vi "Dresden R2R Sputter 03.02.2018 IY24.vi"() -> ()   [LabVIEW 2009] (continued)
                        }
                      }
                      n10678 = Or(x=w17426, y=w17430) -> (x .or. y?=w17427:bool)
                    }
                  }
                  frame #5 {
                    n10679 = local write "Test_stop"(TRUE ("Test_stop")) -> ()
                    n10680 = Wait (ms)(milliseconds to wait=u32 10) -> ()  [unwired: 1 out]
                  }
                }
              }
              frame #1 {
                n10681 = stacked-sequence {
                  tunnel: w17459 -> [_ _ _ _ w17470 _]
                  frame #0 {
                    n10682 = local read "Output voltage value"() -> (w17460:dbl)
                    n10683 = local write "Ch3_SRV_counterclockwise_direction_do"(FALSE ("Ch2_SRV1_direction_do")) -> ()
                    n10684 = local write "Actual Lap"(0.0 ("Actual Lap")) -> ()
                    n10685 = local write "Actual Length"(0.0 ("Actual Region")) -> ()
                    n10686 = Wait (ms)(milliseconds to wait=u32 10) -> ()  [unwired: 1 out]
                    n10687 = local write "Tension_controller1_set_value"(w17460) -> ()
                  }
                  frame #1 {
                    n10688 = local write "Tension_controller1_set"(TRUE ("Tension_controller2_set")) -> ()
                  }
                  frame #2 {
                    n10689 = Wait (ms)(milliseconds to wait=u32 10) -> ()  [unwired: 1 out]
                  }
                  frame #3 {
                    n10690 = local write "Tension_controllers_start/stop_do"(TRUE ("Tension_controllers_start/stop_do")) -> ()
                    n10691 = local write "Ch3_SRV_start_stop_do"(TRUE ("Ch2_SRV1_start_stop_do")) -> ()
                    n10692 = Wait (ms)(milliseconds to wait=u32 10) -> ()  [unwired: 1 out]
                  }
                  frame #4 {
                    n10693 = while {
                      tunnel: w17470 -> [w17472]
                      stop <- w17474 stop-if-true
                      n10694 = Wait Until Next ms Multiple(millisecond multiple=u32 10) -> ()  [unwired: 1 out]
                      n10695 = call "Elapsed Time153"("Reset"=w17472) -> ("Elapsed Time (s)"=w17476:dbl)  [unwired: 11 in, 7 out]
                      "Elapsed Time (s) 10" <- w17476
                      n10696 = case shown="True" FALSE {
                        frame #0 {
                          n10697 = local read "To Left Volt"() -> (w17481:dbl)
                          n10698 = local write "Tension_controller1_set"(TRUE ("Tension_controller2_set")) -> ()
                          n10699 = local write "Tension_controller1_set_value"(w17481) -> ()
                        }
                        frame #1 {
                          n10700 = stacked-sequence {
                            frame #0 {
                              n10701 = local read "Actual Diameter"() -> (w17489:dbl)
                              n10702 = local read "Actual Diameter"() -> (w17486:dbl)
                              n10703 = local read "Web Thickness"() -> (w17495:dbl)
                              n10704 = local read "Actual Lap"() -> (w17487:dbl)
                              n10705 = Increment(x=w17487) -> (x+1=w17485:dbl)
                              n10706 = local read "Actual Length"() -> (w17488:dbl)
                              n10707 = Multiply(x=w17495, y=0.002) -> (x*y=w17496:dbl)
                              n10708 = Multiply(x=w17489, y=3.14) -> (x*y=w17491:dbl)
                              n10709 = local write "Actual Lap"(w17485) -> ()
                              n10710 = Add(x=w17486, y=w17496) -> (x+y=w17494:dbl)
                              n10711 = Divide(x=w17491, y=1000.0) -> (x/y=w17493:dbl)
                              n10712 = local write "Actual Diameter"(w17494) -> ()
                              n10713 = Add(x=w17493, y=w17488) -> (x+y=w17484:dbl)
                              n10714 = disable-structure shown="Disabled" {
                                frame #0 {
                                n10715 = local read "Output voltage value"() -> (w17500:dbl)
                                n10716 = local read "Set voltage value"() -> (w17499:dbl)
                                n10717 = Subtract(x=w17500, y=w17499) -> (x-y=w17498:dbl)
                                n10718 = local write "Output voltage value"(w17498) -> ()
                                }
                                frame #1 {
                                }
                              }
                              n10719 = local write "Actual Length"(w17484) -> ()
                              n10720 = Wait (ms)(milliseconds to wait=u32 10) -> ()  [unwired: 1 out]
                            }
                            frame #1 {
                              n10721 = local read "Output voltage value"() -> (w17501:dbl)
                              n10722 = local write "Tension_controller1_set_value"(w17501) -> ()
                              n10723 = Wait (ms)(milliseconds to wait=u32 10) -> ()  [unwired: 1 out]
                            }
                            frame #2 {
                              n10724 = local write "Tension_controller1_set"(TRUE ("Tension_controller2_set")) -> ()
                              "Actual Region led 5" <- TRUE ("Actual Region")
                            }
                          }
                        }
                      }
                      n10725 = Greater Or Equal?(x=w17476, y="Right to Left 5") -> (x >= y?=w17473:bool)
                      n10726 = local read "Start_roll"() -> (w17479:bool)
                      n10727 = Not(x=w17479) -> (.not. x?=w17477:bool)
                      n10728 = Or(x=w17473, y=w17477) -> (x .or. y?=w17474:bool)
                      n10729 = case shown="True" w17473 {
                        frame #0 {
                        }
                        frame #1 {
                          n10730 = local write "Ch3_SRV_start_stop_do"(FALSE ("Ch2_SRV1_start_stop_do")) -> ()
                        }
                      }
                    }
                  }
                  frame #5 {
                    n10731 = local write "Test_stop"(TRUE ("Test_stop")) -> ()
                    n10732 = Wait (ms)(milliseconds to wait=u32 10) -> ()  [unwired: 1 out]
                  }
                }
              }
            }
          }
          frame #4 {
            n10733 = local read "Roll_side_select"() -> (w17508:enum32{"Left to Right", "Right to Left"})
            n10734 = case shown="\"Left to Right\", Default" w17508 {
              tunnel: w17507 -> [_ w17556]
              tunnel: w17507 -> [w17509 _]
              frame #0 {
                n10735 = stacked-sequence {
                  tunnel: w17509 -> [_ _ _ _ w17520 _]
                  frame #0 {
                    n10736 = local read "Output voltage value"() -> (w17512:dbl)
                    n10737 = local write "Ch4_SRV_counterclockwise_direction_do"(TRUE ("Ch2_SRV1_direction_do")) -> ()
                    n10738 = local write "Actual Lap"(0.0 ("Actual Lap")) -> ()
                    n10739 = local write "Actual Length"(0.0 ("Actual Region")) -> ()
                    n10740 = Wait (ms)(milliseconds to wait=u32 10) -> ()  [unwired: 1 out]
                    n10741 = local write "Tension_controller2_set_value"(w17512) -> ()
                  }
                  frame #1 {
                    n10742 = local write "Tension_controller2_set"(TRUE ("Tension_controller2_set")) -> ()
                  }
                  frame #2 {
                    n10743 = Wait (ms)(milliseconds to wait=u32 10) -> ()  [unwired: 1 out]
                  }
                  frame #3 {
                    n10744 = local write "Tension_controllers_start/stop_do"(TRUE ("Tension_controllers_start/stop_do")) -> ()
                    n10745 = local write "Ch4_SRV_start_stop_do"(TRUE ("Ch2_SRV1_start_stop_do")) -> ()
                    n10746 = Wait (ms)(milliseconds to wait=u32 10) -> ()  [unwired: 1 out]
                  }
                  frame #4 {
                    n10747 = while {
                      tunnel: w17520 -> [w17522]
                      stop <- w17524 stop-if-true
                      n10748 = call "Elapsed Time147"("Reset"=w17522) -> ("Elapsed Time (s)"=w17526:dbl)  [unwired: 11 in, 7 out]
                      "Elapsed Time (s) 7" <- w17526
                      n10749 = Wait Until Next ms Multiple(millisecond multiple=u32 10) -> ()  [unwired: 1 out]
                      n10750 = local read "Start_roll"() -> (w17529:bool)
                      n10751 = Greater Or Equal?(x=w17526, y="Left to Right 4") -> (x >= y?=w17523:bool)
                      n10752 = case shown="True" FALSE {
                        frame #0 {
                          n10753 = local read "To Right Volt"() -> (w17531:dbl)
                          n10754 = local write "Tension_controller2_set_value"(w17531) -> ()
                          n10755 = local write "Tension_controller2_set"(TRUE ("Tension_controller2_set")) -> ()
                        }
                        frame #1 {
                          n10756 = stacked-sequence {
                            frame #0 {
                              n10757 = local read "Actual Diameter"() -> (w17538:dbl)
                              n10758 = local read "Web Thickness"() -> (w17545:dbl)
                              n10759 = local read "Actual Diameter"() -> (w17539:dbl)
                              n10760 = local read "Actual Lap"() -> (w17533:dbl)
                              n10761 = Multiply(x=w17545, y=0.002) -> (x*y=w17546:dbl)
                              n10762 = Increment(x=w17533) -> (x+1=w17534:dbl)
                              n10763 = Add(x=w17538, y=w17546) -> (x+y=w17544:dbl)
                              n10764 = local read "Actual Length"() -> (w17535:dbl)
                              n10765 = Multiply(x=w17539, y=3.14) -> (x*y=w17541:dbl)
                              n10766 = local write "Actual Diameter"(w17544) -> ()
                              n10767 = local write "Actual Lap"(w17534) -> ()
                              n10768 = Divide(x=w17541, y=1000.0) -> (x/y=w17543:dbl)
                              n10769 = Add(x=w17543, y=w17535) -> (x+y=w17536:dbl)
                              n10770 = disable-structure shown="Disabled" {
                                frame #0 {
                                n10771 = local read "Output voltage value"() -> (w17550:dbl)
                                n10772 = local read "Set voltage value"() -> (w17549:dbl)
                                n10773 = Subtract(x=w17550, y=w17549) -> (x-y=w17548:dbl)
                                n10774 = local write "Output voltage value"(w17548) -> ()
                                }
                                frame #1 {
                                }
                              }
                              n10775 = Wait (ms)(milliseconds to wait=u32 10) -> ()  [unwired: 1 out]
                              n10776 = local write "Actual Length"(w17536) -> ()
                            }
                            frame #1 {
                              n10777 = local read "Output voltage value"() -> (w17551:dbl)
                              n10778 = Wait (ms)(milliseconds to wait=u32 10) -> ()  [unwired: 1 out]
                              n10779 = local write "Tension_controller2_set_value"(w17551) -> ()
                            }
                            frame #2 {
                              n10780 = local write "Tension_controller2_set"(TRUE ("Tension_controller2_set")) -> ()
                            }
                          }
                        }
                      }
                      n10781 = Not(x=w17529) -> (.not. x?=w17527:bool)
                      n10782 = case shown="True" w17523 {
                        frame #0 {
                        }
                        frame #1 {
                          n10783 = local write "Ch4_SRV_start_stop_do"(FALSE ("Ch2_SRV1_start_stop_do")) -> ()
                        }
                      }
                      n10784 = Or(x=w17523, y=w17527) -> (x .or. y?=w17524:bool)
                    }
                  }
                  frame #5 {
                    n10785 = local write "Test_stop"(TRUE ("Test_stop")) -> ()
                    n10786 = Wait (ms)(milliseconds to wait=u32 10) -> ()  [unwired: 1 out]
                  }
                }
              }
              frame #1 {
                n10787 = stacked-sequence {
                  tunnel: w17556 -> [_ _ _ _ w17567 _]
                  frame #0 {
                    n10788 = local read "Output voltage value"() -> (w17557:dbl)
                    n10789 = local write "Ch4_SRV_counterclockwise_direction_do"(FALSE ("Ch2_SRV1_direction_do")) -> ()
                    n10790 = local write "Actual Lap"(0.0 ("Actual Lap")) -> ()
                    n10791 = local write "Actual Length"(0.0 ("Actual Region")) -> ()
                    n10792 = Wait (ms)(milliseconds to wait=u32 10) -> ()  [unwired: 1 out]
                    n10793 = local write "Tension_controller1_set_value"(w17557) -> ()
                  }
                  frame #1 {
                    n10794 = local write "Tension_controller1_set"(TRUE ("Tension_controller2_set")) -> ()
                  }
                  frame #2 {
                    n10795 = Wait (ms)(milliseconds to wait=u32 10) -> ()  [unwired: 1 out]
                  }
                  frame #3 {
                    n10796 = local write "Tension_controllers_start/stop_do"(TRUE ("Tension_controllers_start/stop_do")) -> ()
                    n10797 = local write "Ch4_SRV_start_stop_do"(TRUE ("Ch2_SRV1_start_stop_do")) -> ()
                    n10798 = Wait (ms)(milliseconds to wait=u32 10) -> ()  [unwired: 1 out]
                  }
                  frame #4 {
                    n10799 = while {
                      tunnel: w17567 -> [w17569]
                      stop <- w17571 stop-if-true
                      n10800 = Wait Until Next ms Multiple(millisecond multiple=u32 10) -> ()  [unwired: 1 out]
                      n10801 = call "Elapsed Time148"("Reset"=w17569) -> ("Elapsed Time (s)"=w17573:dbl)  [unwired: 11 in, 7 out]
                      "Elapsed Time (s) 8" <- w17573
                      n10802 = case shown="True" FALSE {
                        frame #0 {
                          n10803 = local read "To Left Volt"() -> (w17578:dbl)
                          n10804 = local write "Tension_controller1_set"(TRUE ("Tension_controller2_set")) -> ()
                          n10805 = local write "Tension_controller1_set_value"(w17578) -> ()
                        }
                        frame #1 {
                          n10806 = stacked-sequence {
                            frame #0 {
                              n10807 = local read "Actual Diameter"() -> (w17586:dbl)
                              n10808 = local read "Actual Diameter"() -> (w17583:dbl)
                              n10809 = local read "Web Thickness"() -> (w17592:dbl)
                              n10810 = local read "Actual Lap"() -> (w17584:dbl)
                              n10811 = Increment(x=w17584) -> (x+1=w17582:dbl)
                              n10812 = local read "Actual Length"() -> (w17585:dbl)
                              n10813 = Multiply(x=w17592, y=0.002) -> (x*y=w17593:dbl)
                              n10814 = Multiply(x=w17586, y=3.14) -> (x*y=w17588:dbl)
                              n10815 = local write "Actual Lap"(w17582) -> ()
                              n10816 = Add(x=w17583, y=w17593) -> (x+y=w17591:dbl)
                              n10817 = Divide(x=w17588, y=1000.0) -> (x/y=w17590:dbl)
                              n10818 = local write "Actual Diameter"(w17591) -> ()
                              n10819 = Add(x=w17590, y=w17585) -> (x+y=w17581:dbl)
                              n10820 = disable-structure shown="Disabled" {
                                frame #0 {
                                n10821 = local read "Output voltage value"() -> (w17597:dbl)
                                n10822 = local read "Set voltage value"() -> (w17596:dbl)
                                n10823 = Subtract(x=w17597, y=w17596) -> (x-y=w17595:dbl)
                                n10824 = local write "Output voltage value"(w17595) -> ()
                                }
                                frame #1 {
                                }
                              }
                              n10825 = local write "Actual Length"(w17581) -> ()
                              n10826 = Wait (ms)(milliseconds to wait=u32 10) -> ()  [unwired: 1 out]
                            }
                            frame #1 {
                              n10827 = local read "Output voltage value"() -> (w17598:dbl)
                              n10828 = local write "Tension_controller1_set_value"(w17598) -> ()
                              n10829 = Wait (ms)(milliseconds to wait=u32 10) -> ()  [unwired: 1 out]
                            }
                            frame #2 {
                              n10830 = local write "Tension_controller1_set"(TRUE ("Tension_controller2_set")) -> ()
                              "Actual Region led 4" <- TRUE ("Actual Region")
                            }
                          }
                        }
                      }
                      n10831 = Greater Or Equal?(x=w17573, y="Right to Left 4") -> (x >= y?=w17570:bool)
                      n10832 = local read "Start_roll"() -> (w17576:bool)
                      n10833 = Not(x=w17576) -> (.not. x?=w17574:bool)
                      n10834 = Or(x=w17570, y=w17574) -> (x .or. y?=w17571:bool)
                      n10835 = case shown="True" w17570 {
                        frame #0 {
                        }
                        frame #1 {
                          n10836 = local write "Ch4_SRV_start_stop_do"(FALSE ("Ch2_SRV1_start_stop_do")) -> ()
                        }
                      }
                    }
                  }
                  frame #5 {
                    n10837 = local write "Test_stop"(TRUE ("Test_stop")) -> ()
                    n10838 = Wait (ms)(milliseconds to wait=u32 10) -> ()  [unwired: 1 out]
                  }
                }
              }
            }
          }
        }
      }
    }
  }
  n10839 = while {
    stop <- FALSE stop-if-true
    n10840 = Wait Until Next ms Multiple(millisecond multiple=u32 300) -> ()  [unwired: 1 out]
    n10841 = case shown="True" "Automatic Roll" {
      tunnel: "Auto_roll_ch_select" -> [_ w17608]
      frame #0 {
      }
      frame #1 {
        n10842 = stacked-sequence {
          tunnel: w17608 -> [_ _ _ _ _ w17629 _ _ _ _ _ _ _ _ _ _ _]
          frame #0 {
            n10843 = local write "Calculate_auto"(TRUE ("Calculate_auto")) -> ()
            n10844 = Wait (ms)(milliseconds to wait=u32 100) -> ()  [unwired: 1 out]
          }
          frame #1 {
            n10845 = while {
              stop <- w17611 stop-if-true
              n10846 = local read "Automatic Roll"() -> (w17614:bool)
              n10847 = local read "Calculate_auto"() -> (w17616:bool)
              n10848 = Wait Until Next ms Multiple(millisecond multiple=u32 100 ("milliseconds to wait")) -> ()  [unwired: 1 out]
              n10849 = local read "Semi"() -> (w17612:bool)
              n10850 = Not(x=w17614) -> (.not. x?=w17613:bool)
              n10851 = Not(x=w17616) -> (.not. x?=w17615:bool)
              n10852 = Compound Arithmetic op=OR(w17615, w17613, w17612) -> (w17611:bool)
            }
          }
          frame #2 {
            n10853 = local write "Roll_side_select"(enum32{"Left to Right", "Right to Left"}."Left to Right" ("Roll_side_select")) -> ()
            n10854 = Wait (ms)(milliseconds to wait=u32 100) -> ()  [unwired: 1 out]
          }
          frame #3 {
            n10855 = Wait (ms)(milliseconds to wait=u32 100) -> ()  [unwired: 1 out]
            n10856 = local write "Parameters_auto_set"(TRUE ("Calculate_auto")) -> ()
          }
          frame #4 {
            n10857 = while {
              stop <- w17622 stop-if-true
              n10858 = local read "Parameters_auto_set"() -> (w17627:bool)
              n10859 = local read "Automatic Roll"() -> (w17625:bool)
              n10860 = Wait Until Next ms Multiple(millisecond multiple=u32 100 ("milliseconds to wait")) -> ()  [unwired: 1 out]
              n10861 = local read "Semi"() -> (w17623:bool)
              n10862 = Not(x=w17625) -> (.not. x?=w17624:bool)
              n10863 = Not(x=w17627) -> (.not. x?=w17626:bool)
              n10864 = Compound Arithmetic op=OR(w17626, w17624, w17623) -> (w17622:bool)
            }
          }
          frame #5 {
            n10865 = local write "Target Chamber Sensor"(w17629) -> ()
            n10866 = Wait (ms)(milliseconds to wait=u32 100) -> ()  [unwired: 1 out]
          }
          frame #6 {
            n10867 = Wait (ms)(milliseconds to wait=u32 100) -> ()  [unwired: 1 out]
            n10868 = local write "Start_roll"(TRUE ("Calculate_auto")) -> ()
          }
          frame #7 {
            n10869 = while {
              stop <- w17633 stop-if-true
              n10870 = local read "Start_roll"() -> (w17638:bool)
              n10871 = local read "Automatic Roll"() -> (w17636:bool)
              n10872 = Wait Until Next ms Multiple(millisecond multiple=u32 100 ("milliseconds to wait")) -> ()  [unwired: 1 out]
              n10873 = local read "Semi"() -> (w17634:bool)
              n10874 = Not(x=w17636) -> (.not. x?=w17635:bool)
              n10875 = Not(x=w17638) -> (.not. x?=w17637:bool)
              n10876 = Compound Arithmetic op=OR(w17637, w17635, w17634) -> (w17633:bool)
            }
          }
          frame #8 {
            n10877 = Wait (ms)(milliseconds to wait=u32 2500) -> ()  [unwired: 1 out]
          }
          frame #9 {
            n10878 = local write "Calculate_auto"(TRUE ("Calculate_auto")) -> ()
            n10879 = Wait (ms)(milliseconds to wait=u32 100) -> ()  [unwired: 1 out]
          }
          frame #10 {
            n10880 = while {
              stop <- w17643 stop-if-true
              n10881 = local read "Automatic Roll"() -> (w17646:bool)
              n10882 = local read "Calculate_auto"() -> (w17648:bool)
              n10883 = Wait Until Next ms Multiple(millisecond multiple=u32 100 ("milliseconds to wait")) -> ()  [unwired: 1 out]
              n10884 = local read "Semi"() -> (w17644:bool)
              n10885 = Not(x=w17646) -> (.not. x?=w17645:bool)
              n10886 = Not(x=w17648) -> (.not. x?=w17647:bool)
              n10887 = Compound Arithmetic op=OR(w17647, w17645, w17644) -> (w17643:bool)
            }
          }
          frame #11 {
            n10888 = local write "Roll_side_select"(enum32{"Left to Right", "Right to Left"}."Right to Left" ("Roll_side_select")) -> ()
            n10889 = Wait (ms)(milliseconds to wait=u32 100) -> ()  [unwired: 1 out]
          }
          frame #12 {
            n10890 = Wait (ms)(milliseconds to wait=u32 100) -> ()  [unwired: 1 out]
            n10891 = local write "Parameters_auto_set"(TRUE ("Calculate_auto")) -> ()
          }
          frame #13 {
            n10892 = while {
              stop <- w17654 stop-if-true
              n10893 = local read "Parameters_auto_set"() -> (w17659:bool)
              n10894 = local read "Automatic Roll"() -> (w17657:bool)
              n10895 = Wait Until Next ms Multiple(millisecond multiple=u32 100 ("milliseconds to wait")) -> ()  [unwired: 1 out]
              n10896 = local read "Semi"() -> (w17655:bool)
              n10897 = Not(x=w17657) -> (.not. x?=w17656:bool)
              n10898 = Not(x=w17659) -> (.not. x?=w17658:bool)
              n10899 = Compound Arithmetic op=OR(w17658, w17656, w17655) -> (w17654:bool)
            }
          }
          frame #14 {
            n10900 = Wait (ms)(milliseconds to wait=u32 100) -> ()  [unwired: 1 out]
            n10901 = local write "Start_roll"(TRUE ("Calculate_auto")) -> ()
          }
          frame #15 {
            n10902 = while {
              stop <- w17663 stop-if-true
              n10903 = local read "Start_roll"() -> (w17668:bool)
              n10904 = local read "Automatic Roll"() -> (w17666:bool)
              n10905 = Wait Until Next ms Multiple(millisecond multiple=u32 100 ("milliseconds to wait")) -> ()  [unwired: 1 out]
              n10906 = local read "Semi"() -> (w17664:bool)
              n10907 = Not(x=w17666) -> (.not. x?=w17665:bool)
              n10908 = Not(x=w17668) -> (.not. x?=w17667:bool)
              n10909 = Compound Arithmetic op=OR(w17667, w17665, w17664) -> (w17663:bool)
            }
          }
          frame #16 {
            n10910 = local read "Auto_roll_completed_cycle"() -> (w17671:dbl)
            n10911 = Increment(x=w17671) -> (x+1=w17670:dbl)
            n10912 = Wait (ms)(milliseconds to wait=u32 2500) -> ()  [unwired: 1 out]
            n10913 = local write "Auto_roll_completed_cycle"(w17670) -> ()
          }
        }
      }
    }
  }
  n10914 = VISA Close(VISA resource name=w798, error in (no error)=w799) -> ()  [unwired: 1 out]
  n10915 = VISA Close(VISA resource name=w811, error in (no error)=w810) -> ()  [unwired: 1 out]
  n10916 = while {
    stop <- i16? 0 stop-if-true
    # "TP STATUTE"
    n10917 = stacked-sequence {
      frame #0 {
        n10918 = local read "after substring"() -> (w17678)
        n10919 = local read "Tp1_speed_gui"() -> (w17675)
        n10920 = String Length(string=w17678) -> (length=w17681)
        n10921 = Not Equal To 0?(x=w17681) -> (x != 0?=w17679)
        n10922 = Greater?(x=w17675, y="Tp_max_speed") -> (0:w17677)
        n10923 = case shown="False" w17677 {
          tunnel: [w17684 "Maximum Speed" ("Tp1_statute 2")] -> w17676
          tunnel: w17679 -> [w17683 _]
          tunnel: w17678 -> [w17682 _]
          frame #0 {
            n10924 = case shown="True" w17683 {
              tunnel: [" No connection!" ("Tp1_statute 2") w17688] -> w17684
              tunnel: w17682 -> [_ w17687]
              frame #0 {
                n10925 = local write "Ch1_Tp_on"(i16? 0 ("Tp_on(ch1)")) -> ()
              }
              frame #1 {
                n10926 = String Subset(string=w17687, length (rest)=i32? 6 ("length (rest)")) -> (substring=w17692)  [unwired: 1 out]
                n10927 = Equal?(x=w17692, y="000000") -> (x = y?=w17689)
                n10928 = case shown="True" w17689 {
                  tunnel: ["Accelarating" ("Tp1_statute 2") w17695] -> w17688
                  frame #0 {
                    w17693 = T/1 ("Tp1_accelarate")
                    n10929 = local write "Ch1_Tp_on"(w17693) -> ()
                    "Tp1_accelarate" <- w17693
                  }
                  frame #1 {
                    n10930 = local read "Tp1_speed_gui"() -> (w17696)
                    n10931 = Equal?(x=w17696, y=data[9B]) -> (x = y?=w17698)
                    n10932 = case shown="False" w17698 {
                      tunnel: ["Decelarating" ("Tp1_statute 2") "Stopped" ("Tp1_statute 2")] -> w17695
                      frame #0 {
                        n10933 = local write "Ch1_Tp_on"(i16? 0 ("Tp_on(ch1)")) -> ()
                        "Tp1_decelarate" <- T/1 ("Tp1_decelarate")
                      }
                      frame #1 {
                        n10934 = local write "Ch1_Tp_on"(i16? 0 ("Tp_on(ch1)")) -> ()
                      }
                    }
                  }
                }
              }
            }
          }
          frame #1 {
            n10935 = local write "Ch1_Tp_on"(T/1 ("Tp1_accelarate")) -> ()
          }
        }
        "Tp1_statute" <- w17676
      }
      frame #1 {
        n10936 = local read "Tp2_speed_gui"() -> (w17706)
        n10937 = local read "after substring 2"() -> (w17709)
        n10938 = String Length(string=w17709) -> (length=w17712)
        n10939 = Not Equal To 0?(x=w17712) -> (x != 0?=w17710)
        n10940 = Greater?(x=w17706, y="Tp2_max_speed") -> (0:w17708)
        n10941 = case shown="False" w17708 {
          tunnel: [w17715 "Maximum Speed" ("Tp1_statute 2")] -> w17707
          tunnel: w17710 -> [w17714 _]
          tunnel: w17709 -> [w17713 _]
          frame #0 {
            n10942 = case shown="True" w17714 {
              tunnel: [" No connection!" ("Tp1_statute 2") w17719] -> w17715
              tunnel: w17713 -> [_ w17718]
              frame #0 {
                n10943 = local write "Ch2_Tp_on"(i16? 0 ("Tp_on(ch1)")) -> ()
              }
              frame #1 {
                n10944 = String Subset(string=w17718, length (rest)=i32? 6 ("length (rest)")) -> (substring=w17723)  [unwired: 1 out]
                n10945 = Equal?(x=w17723, y="000000") -> (x = y?=w17720)
                n10946 = case shown="True" w17720 {
                  tunnel: ["Accelarating" ("Tp1_statute 2") w17726] -> w17719
                  frame #0 {
                    w17724 = T/1 ("Tp1_accelarate")
                    n10947 = local write "Ch2_Tp_on"(w17724) -> ()
                    "Tp2_accelarate" <- w17724
                  }
                  frame #1 {
                    n10948 = local read "Tp2_speed_gui"() -> (w17728)
                    n10949 = Equal?(x=w17728, y=data[9B]) -> (x = y?=w17727)
                    n10950 = case shown="False" w17727 {
                      tunnel: ["Decelarating" ("Tp1_statute 2") "Stopped" ("Tp1_statute 2")] -> w17726
                      frame #0 {
                        n10951 = local write "Ch2_Tp_on"(i16? 0 ("Tp_on(ch1)")) -> ()
                        "Tp2_decelarate" <- T/1 ("Tp1_decelarate")
                      }
                      frame #1 {
                        n10952 = local write "Ch2_Tp_on"(i16? 0 ("Tp_on(ch1)")) -> ()
                      }
                    }
                  }
                }
              }
            }
          }
          frame #1 {
            n10953 = local write "Ch2_Tp_on"(T/1 ("Tp_on(ch1)")) -> ()
          }
        }
        "Tp2_statute" <- w17707
      }
      frame #2 {
        n10954 = local read "after substring 3"() -> (w17741)
        n10955 = local read "Tp3_speed_gui"() -> (w17737)
        n10956 = String Length(string=w17741) -> (length=w17743)
        n10957 = Not Equal To 0?(x=w17743) -> (x != 0?=w17742)
        n10958 = Greater?(x=w17737, y="Tp3_max_speed") -> (0:w17740)
        n10959 = case shown="False" w17740 {
          tunnel: [w17746 "Maximum Speed" ("Tp1_statute 2")] -> w17739
          tunnel: w17742 -> [w17745 _]
          tunnel: w17741 -> [w17744 _]
          frame #0 {
            n10960 = case shown="True" w17745 {
              tunnel: [" No connection!" ("Tp1_statute 2") w17750] -> w17746
              tunnel: w17744 -> [_ w17749]
              frame #0 {
                n10961 = local write "Ch3_Tp_on"(i16? 0 ("Tp_on(ch1)")) -> ()
              }
              frame #1 {
                n10962 = String Subset(string=w17749, length (rest)=i32? 6 ("length (rest)")) -> (substring=w17754)  [unwired: 1 out]
                n10963 = Equal?(x=w17754, y="000000") -> (x = y?=w17751)
                n10964 = case shown="True" w17751 {
                  tunnel: ["Accelarating" ("Tp1_statute 2") w17757] -> w17750
                  frame #0 {
                    w17755 = T/1 ("Tp1_accelarate")
                    n10965 = local write "Ch3_Tp_on"(w17755) -> ()
                    "Tp3_accelarate" <- w17755
                  }
                  frame #1 {
                    n10966 = local read "Tp3_speed_gui"() -> (w17759)
                    n10967 = Equal?(x=w17759, y=data[9B]) -> (x = y?=w17758)
                    n10968 = case shown="False" w17758 {
                      tunnel: ["Decelarating" ("Tp1_statute 2") "Stopped" ("Tp1_statute 2")] -> w17757
                      frame #0 {
                        n10969 = local write "Ch3_Tp_on"(i16? 0 ("Tp_on(ch1)")) -> ()
                        "Tp3_decelarate" <- T/1 ("Tp1_decelarate")
                      }
                      frame #1 {
                        n10970 = local write "Ch3_Tp_on"(i16? 0 ("Tp_on(ch1)")) -> ()
                      }
                    }
                  }
                }
              }
            }
          }
          frame #1 {
            n10971 = local write "Ch3_Tp_on"(T/1 ("Tp1_accelarate")) -> ()
          }
        }
        "Tp3_statute" <- w17739
      }
      frame #3 {
        n10972 = local read "Turbo_pump_speed 4"() -> (w17772)
        n10973 = local read "after substring 4"() -> (w17770)
        n10974 = String Length(string=w17770) -> (length=w17774)
        n10975 = Not Equal To 0?(x=w17774) -> (x != 0?=w17771)
        n10976 = Greater?(x=w17772, y="Tp4_max_speed") -> (0:w17769)
        n10977 = case shown="False" w17769 {
          tunnel: [w17777 "Maximum Speed" ("Tp1_statute 2")] -> w17768
          tunnel: w17771 -> [w17776 _]
          tunnel: w17770 -> [w17775 _]
          frame #0 {
            n10978 = case shown="True" w17776 {
              tunnel: [" No connection!" ("Tp1_statute 2") w17781] -> w17777
              tunnel: w17775 -> [_ w17780]
              frame #0 {
                n10979 = local write "Ch4_Tp_on"(i16? 0 ("Tp_on(ch1)")) -> ()
              }
              frame #1 {
                n10980 = String Subset(string=w17780, length (rest)=i32? 6 ("length (rest)")) -> (substring=w17785)  [unwired: 1 out]
                n10981 = Equal?(x=w17785, y="000000") -> (x = y?=w17782)
                n10982 = case shown="False" w17782 {
                  tunnel: ["Accelarating" ("Tp1_statute 2") w17789] -> w17781
                  frame #0 {
                    n10983 = local write "Ch4_Tp_on"(T/1 ("Tp_on(ch1)")) -> ()
                    "Tp4_accelarate" <- T/1 ("Tp1_accelarate")
                  }
                  frame #1 {
                    n10984 = local read "Tp4_speed_gui"() -> (w17791)
                    n10985 = Equal?(x=w17791, y=data[9B]) -> (x = y?=w17790)
                    n10986 = case shown="False" w17790 {
                      tunnel: ["Decelarating" ("Tp1_statute 2") "Stopped" ("Tp1_statute 2")] -> w17789
                      frame #0 {
                        n10987 = local write "Ch4_Tp_on"(i16? 0 ("Tp_on(ch1)")) -> ()
                        "Tp4_decelarate" <- T/1 ("Tp1_decelarate")
                      }
                      frame #1 {
                        n10988 = local write "Ch4_Tp_on"(i16? 0 ("Tp_on(ch1)")) -> ()
                      }
                    }
                  }
                }
              }
            }
          }
          frame #1 {
            n10989 = local write "Ch4_Tp_on"(T/1 ("Tp1_accelarate")) -> ()
          }
        }
        "Tp4_statute" <- w17768
      }
    }
    n10990 = Wait Until Next ms Multiple(millisecond multiple=i32? 300) -> ()  [unwired: 1 out]
  }
  n10991 = VISA Close(VISA resource name=w25, error in (no error)=w24) -> ()  [unwired: 1 out]
  n10992 = VISA Close(VISA resource name=w735, error in (no error)=w734) -> ()  [unwired: 1 out]
  n10993 = VISA Close(VISA resource name=w802, error in (no error)=w801) -> ()  [unwired: 1 out]
  n10994 = VISA Close(VISA resource name=w808, error in (no error)=w807) -> ()  [unwired: 1 out]
  n10995 = VISA Close(VISA resource name=w782, error in (no error)=w781) -> ()  [unwired: 1 out]
  n10996 = while {
    stop <- i16? 0 stop-if-true
    n10997 = local read "Tp1_stop_cmnd"() -> (w17833)
    n10998 = local read "Tp2_stop_cmnd"() -> (w17823)
    n10999 = local read "Tp3_stop_cmnd"() -> (w17815)
    n11000 = local read "Tp4_stop_cmnd"() -> (w17809)
    n11001 = local read "Tp3_statute"() -> (w17801)
    n11002 = Wait Until Next ms Multiple(millisecond multiple=i32? 300) -> ()  [unwired: 1 out]
    n11003 = local read "Tp2_statute"() -> (w17817)
    n11004 = local read "Tp1_statute"() -> (w17824)
    n11005 = local read "Tp4_statute"() -> (w17800)
    n11006 = case shown="True" w17833 {
      tunnel: [w17856 i16? 0] -> w17832
      frame #0 {
        n11007 = local read "Tp1_statute"() -> (w17855)
        n11008 = Equal?(x="Accelarating", y=w17855) -> (x = y?=w17860)
        n11009 = Equal?(x=w17855, y="Maximum Speed") -> (x = y?=w17859)
        n11010 = Or(x=w17860, y=w17859) -> (x .or. y?=w17856)
      }
      frame #1 {
      }
    }
    "TP1_working" <- w17832
    n11011 = Equal?(x="Decelarating", y=w17817) -> (x = y?=w17821)
    n11012 = Equal?(x=w17817, y="Stopped") -> (x = y?=w17816)
    n11013 = case shown="False" w17823 {
      tunnel: [w17849 i16? 0] -> w17822
      frame #0 {
        n11014 = local read "Tp2_statute"() -> (w17848)
        n11015 = Equal?(x="Accelarating", y=w17848) -> (x = y?=w17853)
        n11016 = Equal?(x=w17848, y="Maximum Speed") -> (x = y?=w17852)
        n11017 = Or(x=w17853, y=w17852) -> (x .or. y?=w17849)
      }
      frame #1 {
      }
    }
    "TP2_working" <- w17822
    n11018 = case shown="True" w17815 {
      tunnel: [w17842 i16? 0] -> w17808
      frame #0 {
        n11019 = local read "Tp3_statute"() -> (w17841)
        n11020 = Equal?(x="Accelarating", y=w17841) -> (x = y?=w17846)
        n11021 = Equal?(x=w17841, y="Maximum Speed") -> (x = y?=w17845)
        n11022 = Or(x=w17846, y=w17845) -> (x .or. y?=w17842)
      }
      frame #1 {
      }
    }
    "TP3_working" <- w17808
    n11023 = case shown="False" w17809 {
      tunnel: [w17835 i16? 0] -> w17807
      frame #0 {
        n11024 = local read "Tp4_statute"() -> (w17834)
        n11025 = Equal?(x="Accelarating", y=w17834) -> (x = y?=w17839)
        n11026 = Equal?(x=w17834, y="Maximum Speed") -> (x = y?=w17838)
        n11027 = Or(x=w17839, y=w17838) -> (x .or. y?=w17835)
      }
      frame #1 {
      }
    }
    "TP4_working" <- w17807
    n11028 = Equal?(x="Decelarating", y=w17824) -> (x = y?=w17828)
    n11029 = Equal?(x=w17824, y="Stopped") -> (x = y?=w17829)
    n11030 = Equal?(x="Decelarating", y=w17800) -> (x = y?=w17806)
    n11031 = Equal?(x=w17800, y="Stopped") -> (x = y?=w17805)
    n11032 = Equal?(x="Decelarating", y=w17801) -> (x = y?=w17811)
    n11033 = Equal?(x=w17801, y="Stopped") -> (x = y?=w17812)
    n11034 = Or(x=w17821, y=w17816) -> (x .or. y?=→"Tp2_stopped")
    n11035 = Or(x=w17828, y=w17829) -> (x .or. y?=→"Tp1_stopped")
    n11036 = Or(x=w17806, y=w17805) -> (x .or. y?=→"Tp4_stopped")
    n11037 = Or(x=w17811, y=w17812) -> (x .or. y?=→"Tp3_stopped")
  }
  n11038 = VISA Close(VISA resource name=w743, error in (no error)=w774) -> ()  [unwired: 1 out]
  n11039 = VISA Close(VISA resource name=w744, error in (no error)=w759) -> ()  [unwired: 1 out]
  n11040 = VISA Close(VISA resource name=w757, error in (no error)=w758) -> ()  [unwired: 1 out]
  n11041 = VISA Close(VISA resource name=w745, error in (no error)=w773) -> ()  [unwired: 1 out]
  n11042 = while {
    stop <- FALSE stop-if-true
    n11043 = Wait Until Next ms Multiple(millisecond multiple=u32 300) -> ()  [unwired: 1 out]
    n11044 = Build Array(FALSE, "Transfer_ch1_2", "Transfer_ch2_1", "Transfer_ch2_3", "Transfer_ch3_2", "Transfer_ch3_4", "Transfer_ch4_3") -> (w17870:bool[])
    n11045 = Boolean Array To Number(Boolean array=w17870) -> (number=w17871:u32)
    n11046 = Mantissa & Exponent(0:w17871) -> (2:w17868:dbl)  [unwired: 1 out]
    n11047 = case shown="1" w17868 {
      frame #0 {
      }
      frame #1 {
        n11048 = stacked-sequence {
          frame #0 {
            n11049 = Wait (ms)(milliseconds to wait=u32 1500) -> ()  [unwired: 1 out]
            n11050 = local write "Clean_trnsfr_1_2"(TRUE ("Clean_trnsfr_1_2")) -> ()
            n11051 = local write "system_status"("Chamber 1 to Chamber 2 Transfer Process in Progress." ("system_status")) -> ()
            n11052 = local write "final_process_messages"("Chamber 1 to Chamber 2  Transfer Process was completed." ("final_process_messages")) -> ()
          }
          frame #1 {
            n11053 = stacked-sequence {
              frame #0 {
                n11054 = local write "Routine_check_transfer"(TRUE ("Routine_check_transfer")) -> ()
                n11055 = Wait (ms)(milliseconds to wait=u32 100) -> ()  [unwired: 1 out]
              }
              frame #1 {
                n11056 = while {
                  i -> [w17887]
                  stop <- w17883 stop-if-true
                  n11057 = Greater Or Equal?(x=w17887, y=1500) -> (x >= y?=w17884:bool)
                  n11058 = Wait Until Next ms Multiple(millisecond multiple=u32 200) -> ()  [unwired: 1 out]
                  n11059 = case shown="True" w17884 {
                    frame #0 {
                    }
                    frame #1 {
                      # "Hata mesajı"
                      n11060 = local write "Semi"(TRUE ("Semi")) -> ()
                    }
                  }
                  n11061 = local read "Routine_check_transfer"() -> (w17880:bool)
                  n11062 = local read "Semi"() -> (w17882:bool)
                  n11063 = Not(x=w17880) -> (.not. x?=w17881:bool)
                  n11064 = Or(x=w17881, y=w17882) -> (x .or. y?=w17883:bool)
                }
              }
              frame #2 {
                n11065 = Wait (ms)(milliseconds to wait=u32 500) -> ()  [unwired: 1 out]
              }
            }
          }
          frame #2 {
            # "STARTED UP CH1"
            n11066 = disable-structure shown="Disabled" {
              frame #0 {
                n11067 = local read "Semi"() -> (w17890:bool)
                n11068 = case shown="False" w17890 {
                  frame #0 {
                    n11069 = local read "started_up_ch1"() -> (w17891:bool)
                    n11070 = case shown="False" w17891 {
                      frame #0 {
                        n11071 = stacked-sequence {
                          frame #0 {
                            n11072 = local read "Semi"() -> (w17892:bool)
                            n11073 = case shown="False" w17892 {
                              frame #0 {
                                n11074 = local write "Start_up_ch1"(TRUE ("Start_up_ch2")) -> ()
                              }
                              frame #1 {
                              }
                            }
                          }
                          frame #1 {
                            n11075 = local read "Semi"() -> (w17894:bool)
                            n11076 = case shown="False" w17894 {
                              frame #0 {
                                n11077 = Wait (ms)(milliseconds to wait=u32 16000) -> ()  [unwired: 1 out]
                              }
                              frame #1 {
                              }
                            }
                          }
                          frame #2 {
                            n11078 = local read "Semi"() -> (w17896:bool)
                            n11079 = case shown="False" w17896 {
                              frame #0 {
                                n11080 = while {
                                i -> [w17901]
                                stop <- w17898 stop-if-true
                                n11081 = Greater?(x=w17901, y=80) -> (0:w17899:bool)
                                n11082 = local read "started_up_ch1"() -> (w17897:bool)
                                n11083 = case shown="True" w17899 {
                                frame #0 {
                                }
                                frame #1 {
                                n11084 = local write "Semi"(TRUE ("Semi")) -> ()
                                n11085 = local write "Error Message"("Chamber 1 Pressure is not suitable  \nfor transfer process!\nPlease check connections." ("Error Message")) -> ()
                                }
                                }
                                n11086 = case shown="False" w17897 {
                                tunnel: [FALSE TRUE] -> w17898
                                frame #0 {
                                n11087 = Wait Until Next ms Multiple(millisecond multiple=u32 200) -> ()  [unwired: 1 out]
                                }
                                frame #1 {
                                }
                                }
                                }
                              }
                              frame #1 {
                              }
                            }
                          }
                          frame #3 {
                            n11088 = local read "Semi"() -> (w17907:bool)
                            n11089 = case shown="False" w17907 {
                              frame #0 {
                                n11090 = local write "CH1_2_trns_0"(TRUE ("CH1_2_trns_0")) -> ()
                                n11091 = Wait (ms)(milliseconds to wait=u32 1000) -> ()  [unwired: 1 out]